vi "Derivative of intensity graph-JKI SM.vi"() -> ()   [LabVIEW 2016] (continued)
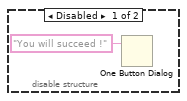
[diagram p2: hidden frame]
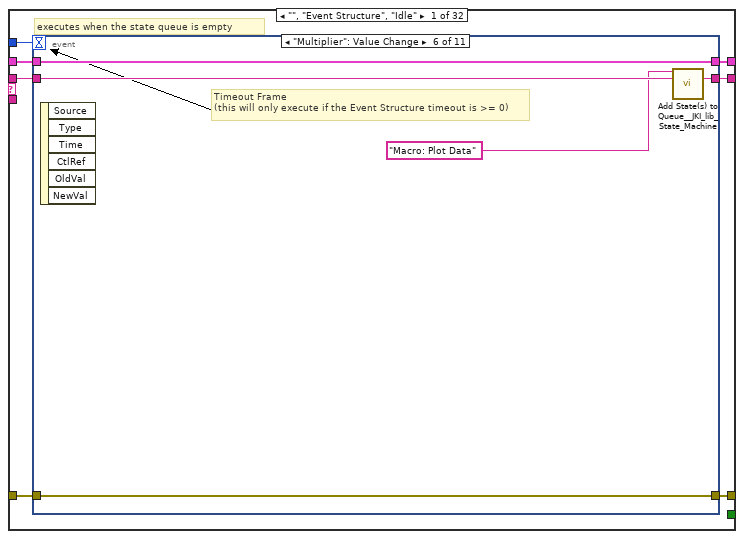
[diagram p3: hidden frame]
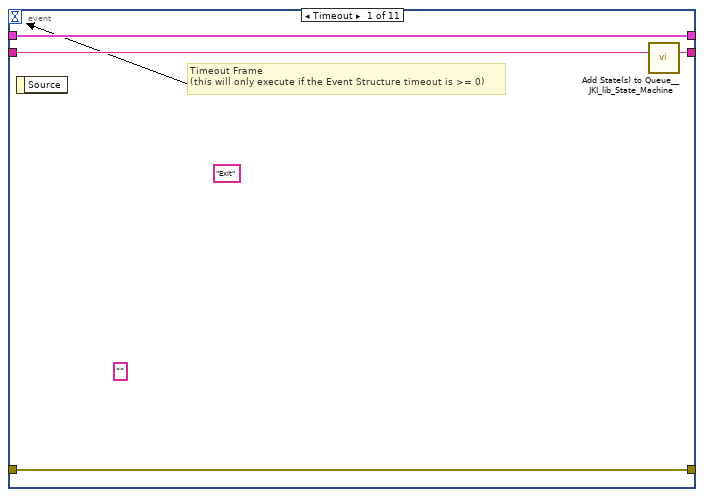
[diagram p4: hidden frame]
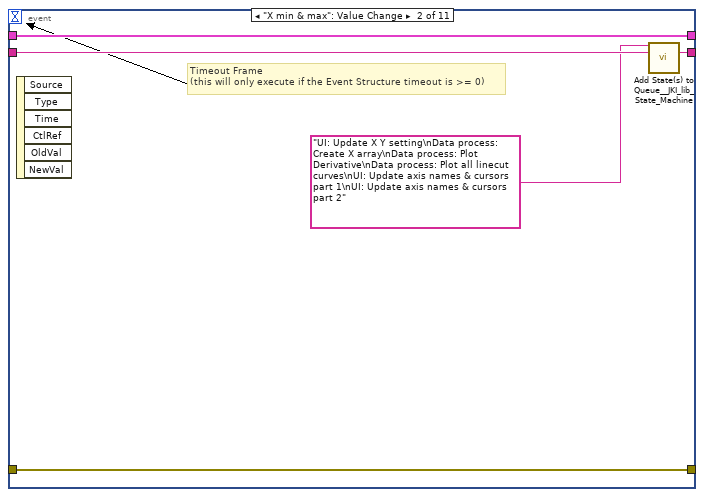
[diagram p5: hidden frame]
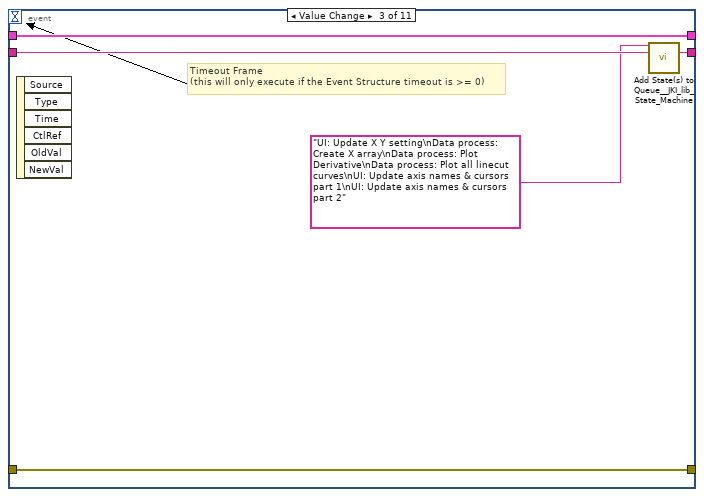
[diagram p6: hidden frame]
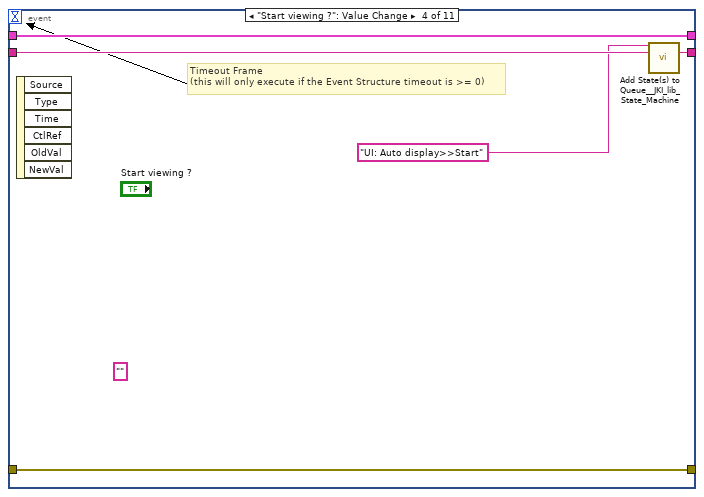
[diagram p7: hidden frame]
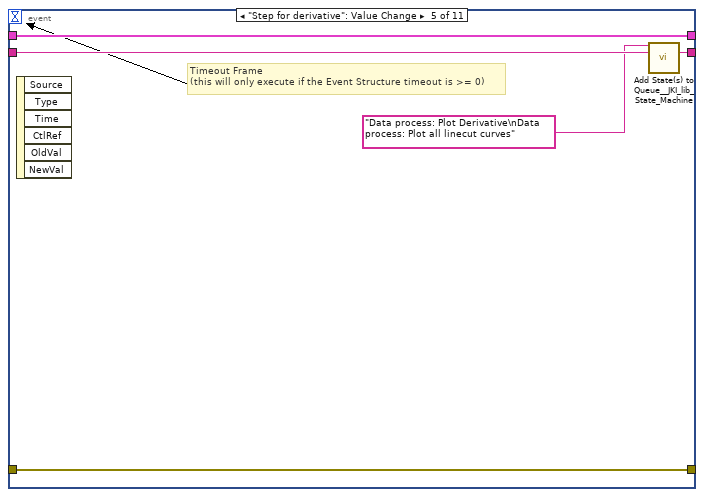
[diagram p8: hidden frame]
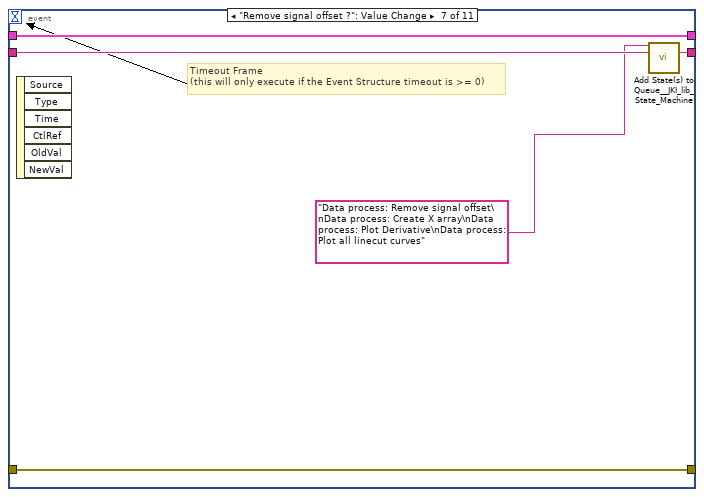
[diagram p9: hidden frame]
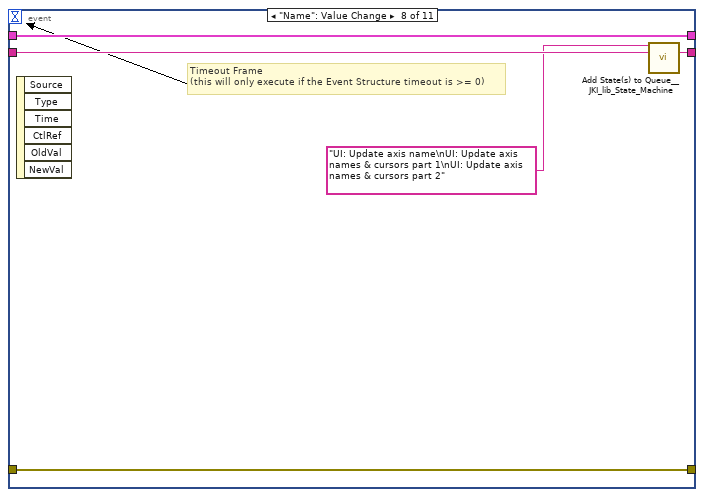
[diagram p10: hidden frame]
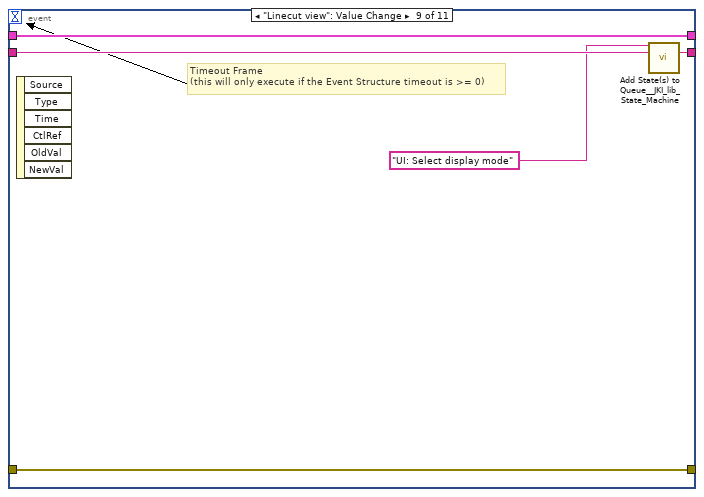
[diagram p11: hidden frame]
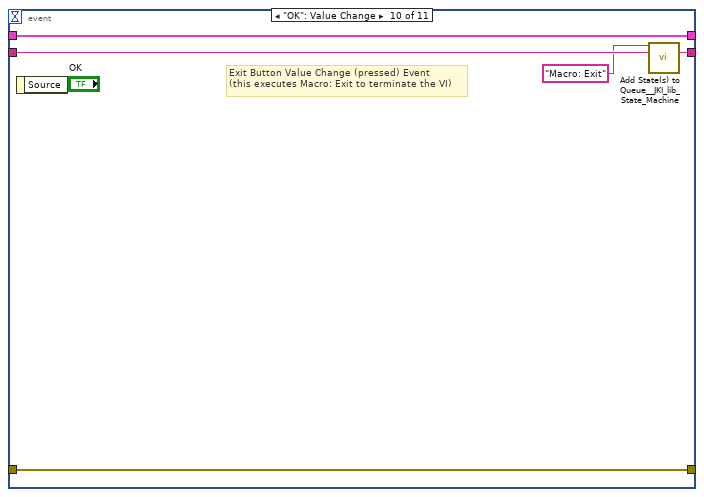
[diagram p12: hidden frame]
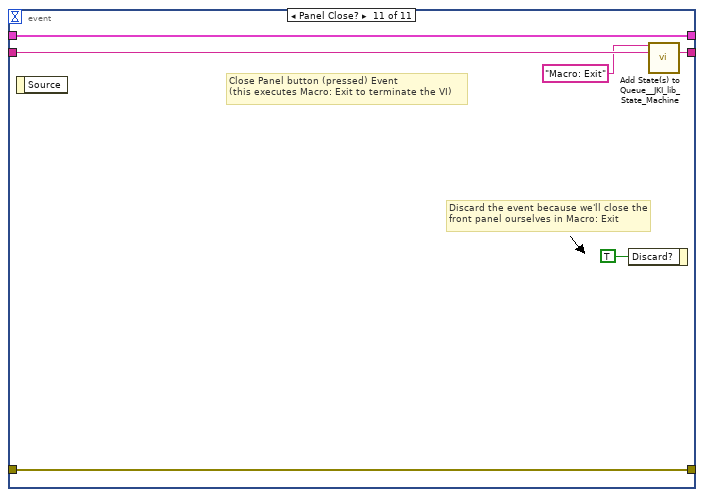
[diagram p13: hidden frame]
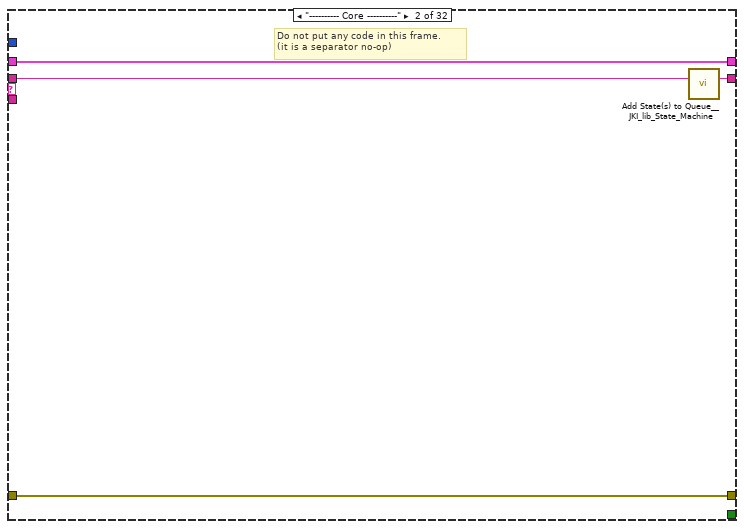
[diagram p14: hidden frame]
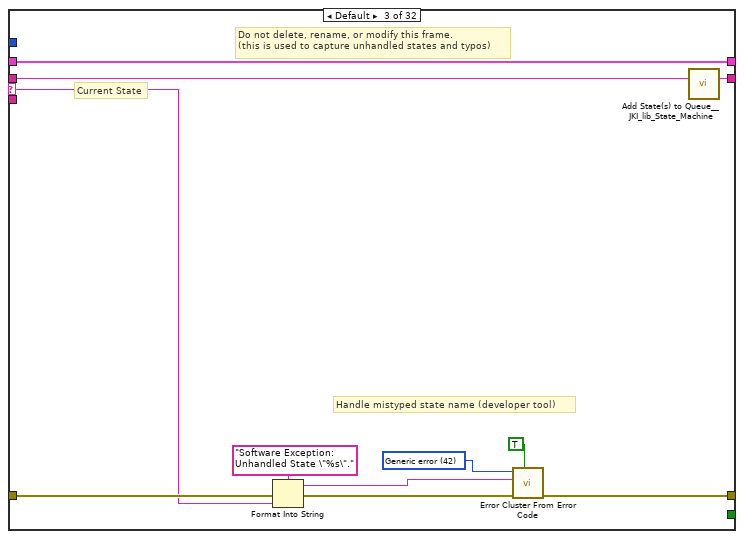
[diagram p15: hidden frame]
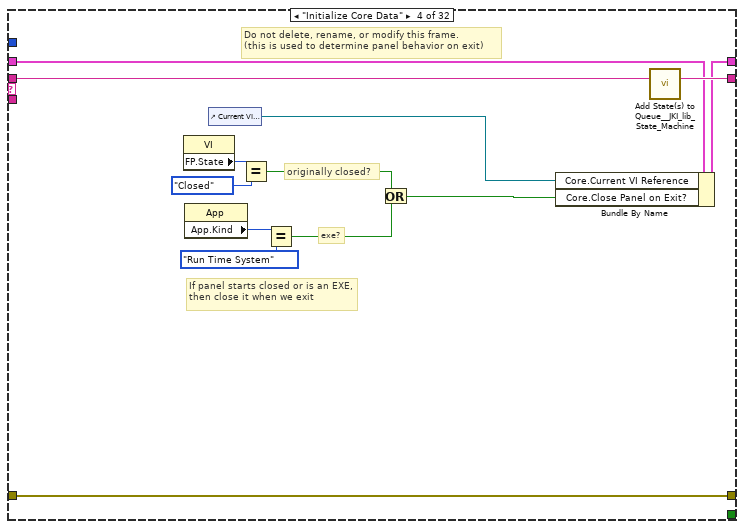
[diagram p16: hidden frame]
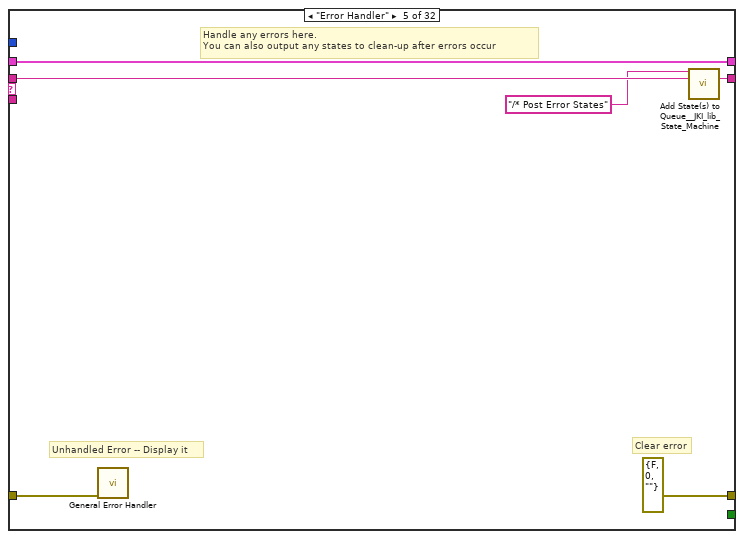
[diagram p17: hidden frame]
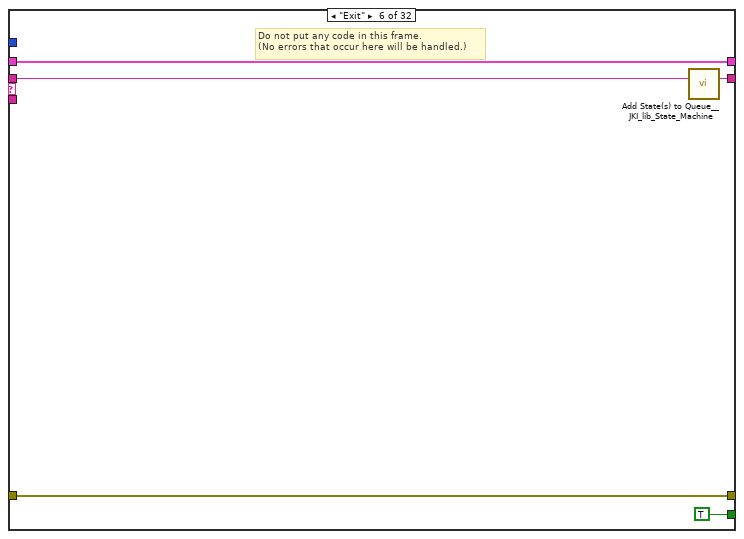
[diagram p18: hidden frame]
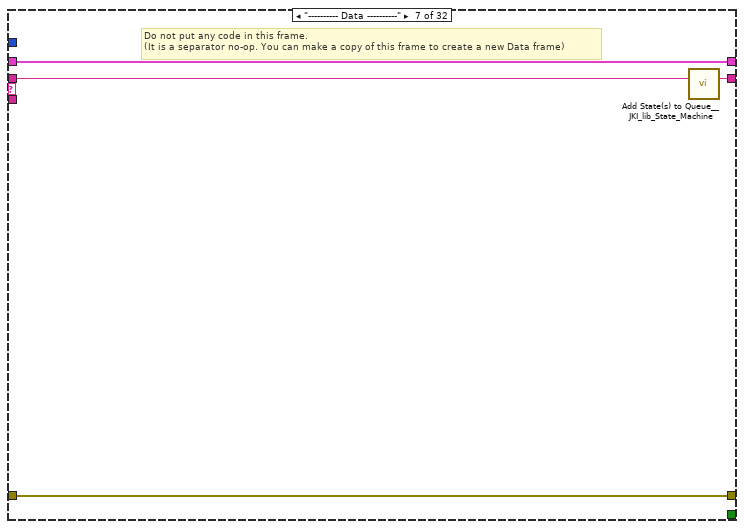
[diagram p19: hidden frame]
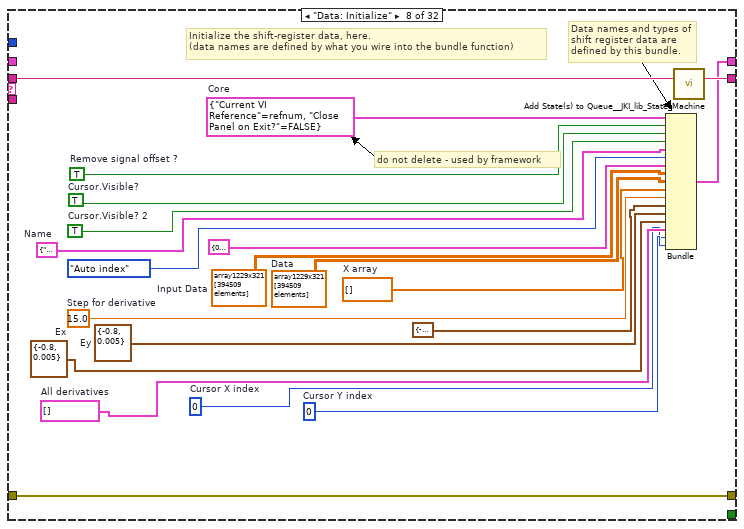
[diagram p20: hidden frame]
        # "Current State"
        # "Do not delete, rename, or modify this frame.\n(this is used to capture unhandled states and typos)"
        # "Handle mistyped state name (developer tool)"
        n30 = Format Into String(format string="Software Exception: Unhandled State \"%s\"." ("message"), error in=w85, w80) -> (resulting string=w88:string, error out=w87:errorcluster)  [unwired: 1 in]
        n31 = call <vilib>:"Error Cluster From Error Code.vi"("show call chain? (False)"=TRUE, "error in (no error)"=w87, "error message (\"\")"=w88, "error code (0)"=w89) -> ("error out"=w86:errorcluster)  [unwired: 5 in]
        n32 = call <vilib>:"Add State(s) to Queue__JKI_lib_State_Machine.vi"("State(s) in (\"\")"=w84) -> ("States Out"=w83:string)  [unwired: 14 in]
      }
      frame "Initialize Core Data" {
        # "Do not delete, rename, or modify this frame.\n(this is used to determine panel behavior on exit)"
        # "originally closed?"
        # "exe?"
        # "If panel starts closed or is an EXE, then close it when we exit"
        n33 = property class="VI"() -> ("FP.State"=w93:T5)  [unwired: 2 in, 2 out]
        n34 = property class="App"() -> ("App.Kind"=w99:T6)  [unwired: 2 in, 2 out]
        n35 = control-ref of="Current VI Reference"() -> (w94:refnum<vi>)
        n36 = Equal?(x=w93, y=T5."Closed" ("Front Panel Window:State")) -> (x = y?=w91:bool)
        n37 = Equal?(x=w99, y=T6."Run Time System" ("Application:Kind")) -> (x = y?=w97:bool)
        n38 = Or(x=w91, y=w97) -> (x .or. y?=w95:bool)
        n39 = Bundle By Name(cluster=w96, "Core.Current VI Reference"=w94, "Core.Close Panel on Exit?"=w95) -> (w101:T7)
        n40 = call <vilib>:"Add State(s) to Queue__JKI_lib_State_Machine.vi"("State(s) in (\"\")"=w103) -> ("States Out"=w102:string)  [unwired: 14 in]
      }
      frame "Error Handler" {
        # "Unhandled Error -- Display it"
        # "Handle any errors here.\nYou can also output any states to clean-up after errors occur"
        # "Clear error"
        n41 = call <vilib>:"General Error Handler.vi"("error in (no error)"=w105) -> ()  [unwired: 10 in, 5 out]
        n42 = call <vilib>:"Add State(s) to Queue__JKI_lib_State_Machine.vi"("State(s) in Front (\"\")"="/* Post Error States", "State(s) in (\"\")"=w109) -> ("States Out"=w108:string)  [unwired: 13 in]
      }
      frame "Exit" {
        # "Do not put any code in this frame.\n(No errors that occur here will be handled.)"
        n43 = call <vilib>:"Add State(s) to Queue__JKI_lib_State_Machine.vi"("State(s) in (\"\")"=w114) -> ("States Out"=w113:string)  [unwired: 14 in]
      }
      frame "---------- Data ----------" {
        # "Do not put any code in this frame.\n(It is a separator no-op. You can make a copy of this frame to create a new Data frame)"
        n44 = call <vilib>:"Add State(s) to Queue__JKI_lib_State_Machine.vi"("State(s) in (\"\")"=w118) -> ("States Out"=w117:string)  [unwired: 14 in]
      }
      frame "Data: Initialize" {
        w120 = T1 {"Offset"=-0.8, "Multiplier"=0.005}  # Ex
        w122 = 0  # Cursor Y index
        w121 = 0  # Cursor X index
        w123 = cluster{dbl[], dbl[]}[] []  # All derivatives
        w124 = dbl[] []  # X array
        w125 = dbl[][] array1229x321[394509 elements]  # Data
        w126 = T1 {"Offset"=-0.8, "Multiplier"=0.005}  # Ey
        w127 = 15.0  # Step for derivative
        w128 = dbl[][] array1229x321[394509 elements]  # Input Data
        w131 = T4 {"X"="Vsd (V)", "Y"="VsgL (V)", "Z"="I (A)", "dZ/dX"="dI/dV (S)"}  # Name
        w132 = TRUE  # Cursor.Visible? 2
        w133 = TRUE  # Cursor.Visible?
        w134 = T8 {"Current VI Reference"=refnum, "Close Panel on Exit?"=FALSE}  # Core
        w135 = TRUE  # Remove signal offset ?
        # "do not delete - used by framework"
        # "Data names and types of shift register data are defined by this bundle."
        # "Initialize the shift-register data, here.\n(data names are defined by what you wire into the bundle function)"
        n45 = Bundle("Core"=w134, "Remove signal offset ?"=w135, "Cursor.Visible?"=w133, "Cursor.Visible? 2"=w132, "Name"=w131, "Linecut view"=enum16{"Manual index", "Auto index"}."Auto index", "Signal offset to Subtract"=T3 {"X value"=0.0, "Y value"=0.0, "X for all Y values ?"=FALSE}, "Input Data"=w128, "Data"=w125, "X array"=w124, "Step for derivative"=w127, "X min & max"=cluster{"X min":dbl, "X max":dbl} {"X min"=-0.1923, "X max"=0.2993}, "Ey"=w126, "Ex"=w120, "All derivatives"=w123, "Cursor X index"=w121, "Cursor Y index"=w122) -> (w137:T7)  [unwired: 1 in]
        n46 = call <vilib>:"Add State(s) to Queue__JKI_lib_State_Machine.vi"("State(s) in (\"\")"=w139) -> ("States Out"=w138:string)  [unwired: 14 in]
      }
      frame "Data: Cleanup" {
        # "Cleanup any data and references, here.\n(this is called automatically, by the Macro: Exit)"
        n47 = Unbundle By Name(w140) -> ("Core.Current VI Reference"=w143:refnum<vi>)
        n48 = Close Reference(reference=w143, error in (no error)=w142) -> (error out=w141:errorcluster)
        n49 = call <vilib>:"Add State(s) to Queue__JKI_lib_State_Machine.vi"("State(s) in (\"\")"=w145) -> ("States Out"=w144:string)  [unwired: 14 in]
      }
      frame "---------- UI ----------" {
        # "Do not put any code in this frame.\n(It is a separator no-op. You can make a copy of this frame to create a new UI frame)"
        n50 = call <vilib>:"Add State(s) to Queue__JKI_lib_State_Machine.vi"("State(s) in (\"\")"=w149) -> ("States Out"=w148:string)  [unwired: 14 in]
      }
      frame "UI: Initialize" {
        # "Initialize the User Interface, here.\n(this is called automatically, by the Macro: Init)"
        n51 = call <vilib>:"Add State(s) to Queue__JKI_lib_State_Machine.vi"("State(s) in (\"\")"=w153) -> ("States Out"=w152:string)  [unwired: 14 in]
      }
      frame "UI: Cursor Set" {
        # "Argument"
        # "Set and Unset Cursor Busy.\n(Usage: \"UI: Cursor Set >> Busy|Idle\")"
        n52 = case shown="\"Idle\", Default" w154 {
          tunnel: w156 -> [w161 w163]
          tunnel: [w160 w162] -> w155
          frame "Idle", Default {
            n53 = call <vilib>:"Unset Busy.vi"("error in (no error)"=w161) -> ("error out"=w160:errorcluster)  [unwired: 10 in]
          }
          frame "Busy" {
            n54 = call <vilib>:"Set Busy.vi"("error in (no error)"=w163) -> ("error out"=w162:errorcluster)  [unwired: 9 in, 1 out]
          }
        }
        n55 = call <vilib>:"Add State(s) to Queue__JKI_lib_State_Machine.vi"("State(s) in (\"\")"=w159) -> ("States Out"=w158:string)  [unwired: 14 in]
      }
      frame "UI: Front Panel State" {
        # "Argument"
        # "Set Front Panel Open or Closed\n(Usage: \"UI: Front Panel State >> Open|Close\")"
        n56 = Unbundle By Name(w166) -> ("Core.Current VI Reference"=w165:refnum<vi>)
        n57 = case shown="\"Open\", \"Standard\", Default" w164 {
          tunnel: w168 -> [w176 w191 w202 w215 w228]
          tunnel: [w178 w192 w204 w217 w230] -> w167
          tunnel: w165 -> [w177 w189 w203 w216 w229]
          frame "Open", "Standard", Default {
            w171 = T5."Standard" ("State")
            n58 = property class="VI"(reference=w177, error in=w176) -> (reference out=w174:refnum<vi>, error out=w175:errorcluster, "FP.State"=w173:T5)
            n59 = Not Equal?(x=w173, y=w171) -> (x != y?=w172:bool)
            n60 = case shown="False" w172 {
              tunnel: [w182 w184] -> w178
              tunnel: w175 -> [w181 w184]
              tunnel: w174 -> [w180 _]
              tunnel: w171 -> [w179 _]
              frame True {
                n61 = invoke class="VI" method="FP.Open"(reference=w180, error in=w181, "Activate"=TRUE, "State"=w179) -> (error out=w182:errorcluster)  [unwired: 1 in, 4 out]
              }
              frame False {
              }
            }
          }
          frame "Close", "Closed" {
            n62 = property class="VI"(reference=w189, error in=w191) -> (reference out=w188:refnum<vi>, error out=w190:errorcluster, "FP.State"=w186:T5)
            n63 = Not Equal?(x=w186, y=T5."Closed" ("Front Panel Window:State")) -> (x != y?=w185:bool)
            n64 = case shown="True" w185 {
              tunnel: [w193 w196] -> w192
              tunnel: w190 -> [w193 w195]
              tunnel: w188 -> [_ w194]
              frame False {
              }
              frame True {
                n65 = invoke class="VI" method="FP.Close"(reference=w194, error in=w195) -> (error out=w196:errorcluster)  [unwired: 1 in, 2 out]
              }
            }
          }
          frame "Hidden", "Hide" {
            w197 = T5."Hidden" ("State")
            n66 = property class="VI"(reference=w203, error in=w202) -> (reference out=w200:refnum<vi>, error out=w201:errorcluster, "FP.State"=w199:T5)
            n67 = Not Equal?(x=w199, y=w197) -> (x != y?=w198:bool)
            n68 = case shown="True" w198 {
              tunnel: [w208 w209] -> w204
              tunnel: w201 -> [w207 w209]
              tunnel: w200 -> [w206 _]
              tunnel: w197 -> [w205 _]
              frame True {
                n69 = invoke class="VI" method="FP.Open"(reference=w206, error in=w207, "State"=w205) -> (error out=w208:errorcluster)  [unwired: 2 in, 4 out]
              }
              frame False {
              }
            }
          }
          frame "Minimize", "Minimized" {
            w210 = T5."Minimized" ("State")
            n70 = property class="VI"(reference=w216, error in=w215) -> (reference out=w213:refnum<vi>, error out=w214:errorcluster, "FP.State"=w212:T5)
            n71 = Not Equal?(x=w212, y=w210) -> (x != y?=w211:bool)
            n72 = case shown="True" w211 {
              tunnel: [w221 w222] -> w217
              tunnel: w214 -> [w220 w222]
              tunnel: w213 -> [w219 _]
              tunnel: w210 -> [w218 _]
              frame True {
                n73 = invoke class="VI" method="FP.Open"(reference=w219, error in=w220, "State"=w218) -> (error out=w221:errorcluster)  [unwired: 2 in, 4 out]
              }
              frame False {
              }
            }
          }
          frame "Maximize", "Maximized" {
            w223 = T5."Maximized" ("State")
            n74 = property class="VI"(reference=w229, error in=w228) -> (reference out=w226:refnum<vi>, error out=w227:errorcluster, "FP.State"=w225:T5)
            n75 = Not Equal?(x=w225, y=w223) -> (x != y?=w224:bool)
            n76 = case shown="True" w224 {
              tunnel: [w234 w235] -> w230
              tunnel: w227 -> [w233 w235]
              tunnel: w226 -> [w232 _]
              tunnel: w223 -> [w231 _]
              frame True {
                n77 = invoke class="VI" method="FP.Open"(reference=w232, error in=w233, "State"=w231) -> (error out=w234:errorcluster)  [unwired: 2 in, 4 out]
              }
              frame False {
              }
            }
          }
        }
        n78 = call <vilib>:"Add State(s) to Queue__JKI_lib_State_Machine.vi"("State(s) in (\"\")"=w170) -> ("States Out"=w169:string)  [unwired: 14 in]
      }
      frame "UI: Set background to Red" {
        # "Do not put any code in this frame.\n(It is a separator no-op. You can make a copy of this frame to create a new UI frame)"
        n79 = Unbundle By Name(w244) -> ("Core.Current VI Reference"=w243:refnum<vi>)
        n80 = property class="VI"(reference=w243) -> ("Panel"=w242:refnum<vi>)  [unwired: 1 in, 2 out]
        n81 = property class="Pnl"(reference=w242) -> (reference out=w241:refnum<vi>, error out=w239:errorcluster, "Panes[]"=w240:refnum<vi>[])  [unwired: 1 in]
        n82 = for {
          tunnel: w240 -> [w250] mode=indexing
          shift-right: [w247] -> w238
          shift-left: w239 -> [w248]
          n83 = property class="Pane"(reference=w250, error in=w248, "PaneColor"=u32 13816530) -> (error out=w247:errorcluster)  [unwired: 1 out]
        }
        n84 = Close Reference(reference=w240, error in (no error)=w238) -> (error out=w237:errorcluster)
        n85 = Close Reference(reference=w241, error in (no error)=w237) -> (error out=w236:errorcluster)
        n86 = call <vilib>:"Add State(s) to Queue__JKI_lib_State_Machine.vi"("State(s) in (\"\")"=w246) -> ("States Out"=w245:string)  [unwired: 14 in]
      }
      frame "UI: Select display mode" {
        # "Do not put any code in this frame.\n(It is a separator no-op. You can make a copy of this frame to create a new UI frame)"
        n87 = case shown="\"Auto index\"" "Linecut view" {
          tunnel: ["UI: Manual display" ("State(s) in Front (\"\")") "UI: Auto display" ("State(s) in Front (\"\")")] -> w251
          frame "Manual index", Default {
          }
          frame "Auto index" {
          }
        }
        n88 = call <vilib>:"Add State(s) to Queue__JKI_lib_State_Machine.vi"("State(s) in Front (\"\")"=w251, "State(s) in (\"\")"=w256) -> ("States Out"=w255:string)  [unwired: 13 in]
      }
      frame "UI: Update X Y setting" {
        # "Do not put any code in this frame.\n(It is a separator no-op. You can make a copy of this frame to create a new UI frame)"
        n89 = Unbundle By Name(w263) -> ("Data"=w265:dbl[][])
        n90 = Transpose 2D Array(2D array=w265) -> (transposed array=w269:dbl[][])
        n91 = Unbundle By Name("X min & max") -> ("X max"=w271:dbl, "X min"=w264:dbl)
        n92 = Array Size(array=w269) -> (size(s)=w268:i32[])
        n93 = Index Array(array=w268) -> (element #2=w267:i32)  [unwired: 2 in, 1 out]
        n94 = Subtract(x=w271, y=w264) -> (x-y=w270:dbl)
        n95 = Divide(x=w270, y=w267) -> (x/y=w266:dbl)
        n96 = Bundle By Name(cluster="Ey", "Multiplier"=w266, "Offset"=w264) -> (w260:T1)
        n97 = Bundle By Name(cluster=w263, "Ey"="Ey", "Ex"=w260, "X min & max"="X min & max") -> (w262:T7)
        n98 = call <vilib>:"Add State(s) to Queue__JKI_lib_State_Machine.vi"("State(s) in (\"\")"=w274) -> ("States Out"=w273:string)  [unwired: 14 in]
      }
      frame "UI: Update axis name" {
        # "Do not put any code in this frame.\n(It is a separator no-op. You can make a copy of this frame to create a new UI frame)"
        n99 = Bundle By Name(cluster=w277, "Name"="Name") -> (w276:T7)
        n100 = call <vilib>:"Add State(s) to Queue__JKI_lib_State_Machine.vi"("State(s) in (\"\")"=w280) -> ("States Out"=w279:string)  [unwired: 14 in]
      }
      frame "UI: Update axis names & cursors part 1" {
        # "Do not put any code in this frame.\n(It is a separator no-op. You can make a copy of this frame to create a new UI frame)"
        n101 = Unbundle By Name(w305) -> ("Name.X"=w287:string, "Name.Y"=w281:string, "Name.Z"=w291:string, "Name.dZ/dX"=w303:string, "Ex"=w292:T1, "Ey"=w297:T1, "Cursor X index"=w302:i32, "Cursor Y index"=w295:i32)
        n102 = Unbundle By Name(w297) -> ("Multiplier"=w296:dbl, "Offset"=w294:dbl)
        n103 = Unbundle By Name(w292) -> ("Multiplier"=w301:dbl, "Offset"=w300:dbl)
        n104 = Multiply(x=w302, y=w301) -> (x*y=w299:dbl)
        n105 = Multiply(x=w295, y=w296) -> (x*y=w298:dbl)
        n106 = Add(x=w300, y=w299) -> (x+y=w289:dbl)
        n107 = Add(x=w294, y=w298) -> (x+y=w284:dbl)
        n108 = Format Into String(format string="= %.1p", w284) -> (resulting string=w282:string)  [unwired: 2 in, 1 out]
        n109 = Concatenate Strings(w281, w282) -> (→"Y value (for X axis)":string)
        n110 = Format Into String(format string="= %.1p", w289) -> (resulting string=w288:string)  [unwired: 2 in, 1 out]
        n111 = Concatenate Strings(w287, w288) -> (→"X value (for Y axis)":string)
        n112 = property on="Data" class="IntGraph (strict)"("Cursor.Cursor X"=w289, "Cursor.Cursor Y"=w284, "XScale.Ofst&Mult"=w292, "YScale.Ofst&Mult"=w297, "Cursor.Visible"="Cursor.Visible ? - Data", "XScale.NameLbl.Text"=w287, "YScale.NameLbl.Text"=w281, "ZScale.NameLbl.Text"=w291) -> ()  [unwired: 2 in, 2 out]
        n113 = property on="Derivative of Data" class="IntGraph (strict)"("Cursor.Cursor X"=w289, "Cursor.Cursor Y"=w284, "XScale.Ofst&Mult"=w292, "YScale.Ofst&Mult"=w297, "Cursor.Visible"="Cursor.Visible ? - Derivative", "XScale.NameLbl.Text"=w287, "YScale.NameLbl.Text"=w281, "ZScale.NameLbl.Text"=w303) -> ()  [unwired: 2 in, 2 out]
        n114 = call <vilib>:"Add State(s) to Queue__JKI_lib_State_Machine.vi"("State(s) in (\"\")"=w308) -> ("States Out"=w307:string)  [unwired: 14 in]
      }
      frame "UI: Update axis names & cursors part 2" {
        # "Do not put any code in this frame.\n(It is a separator no-op. You can make a copy of this frame to create a new UI frame)"
        n115 = Unbundle By Name(w315) -> ("Name.X"=w309:string, "Name.Y"=w313:string, "Name.Z"=w310:string, "Name.dZ/dX"=w314:string, "Ex"=w311:T1, "Ey"=w312:T1)
        n116 = property on="All derivatives" class="XYGraph (strict)"("XScale.NameLbl.Text"=w309, "YScale.NameLbl.Text"=w314) -> ()  [unwired: 2 in, 2 out]
        n117 = property on="Linecut along X axis" class="WFGraph (strict)"("XScale.Ofst&Mult"=w311, "XScale.NameLbl.Text"=w309, "YScale.NameLbl.Text"=w310) -> ()  [unwired: 2 in, 2 out]
        n118 = property on="Linecut along Y axis" class="WFGraph (strict)"("XScale.Ofst&Mult"=w312, "XScale.NameLbl.Text"=w313, "YScale.NameLbl.Text"=w310) -> ()  [unwired: 2 in, 2 out]
        n119 = property on="Linecut of Data 2" class="WFGraph (strict)"("XScale.Ofst&Mult"=w311, "XScale.NameLbl.Text"=w309, "YScale.NameLbl.Text"=w310) -> ()  [unwired: 2 in, 2 out]
        n120 = property on="Linecut of derivative 2" class="XYGraph (strict)"("XScale.NameLbl.Text"=w309, "YScale.NameLbl.Text"=w310) -> ()  [unwired: 2 in, 2 out]
        n121 = property on="Linecut of derivative" class="XYGraph (strict)"("XScale.NameLbl.Text"=w309, "YScale.NameLbl.Text"=w310) -> ()  [unwired: 2 in, 2 out]
        n122 = call <vilib>:"Add State(s) to Queue__JKI_lib_State_Machine.vi"("State(s) in (\"\")"=w318) -> ("States Out"=w317:string)  [unwired: 14 in]
      }
      frame "UI: Manual display" {
        # "Do not put any code in this frame.\n(It is a separator no-op. You can make a copy of this frame to create a new UI frame)"
        n123 = Unbundle By Name(w325) -> ("Data"=w329:dbl[][], "All derivatives"=w321:cluster{dbl[], dbl[]}[])  [unwired: 2 out]
        n124 = Transpose 2D Array(2D array=w329) -> (transposed array=w327:dbl[][])
        n125 = Index Array(array=w327, index (col)="X index (Y axis)") -> (element=→"Linecut along Y axis":dbl[])  [unwired: 1 in]
        n126 = Index Array(array=w321, index="Y index (X axis)") -> (element=→"Linecut of derivative":cluster{dbl[], dbl[]})
        n127 = Index Array(array=w327, index (row)="Y index (X axis)") -> (element=→"Linecut along X axis":dbl[])  [unwired: 1 in]
        n128 = Bundle By Name(cluster=w325, "Cursor X index"="X index (Y axis)", "Cursor Y index"="Y index (X axis)") -> (w324:T7)
        n129 = call <vilib>:"Add State(s) to Queue__JKI_lib_State_Machine.vi"("State(s) in Front (\"\")"="UI: Update axis names & cursors part 1\nEvent Structure//check for UI change\nUI: Manual display" ("State(s) in Front (\"\")"), "State(s) in (\"\")"=w332) -> ("States Out"=w331:string)  [unwired: 13 in]
      }
      frame "UI: Auto display" {
        # "Do not put any code in this frame.\n(It is a separator no-op. You can make a copy of this frame to create a new UI frame)"
        n130 = case shown="\"Increment\"" w336 {
          tunnel: w335 -> [w344 w374 w378 w382]
          tunnel: w338 -> [w345 w377 w379 w383]
          tunnel: [w345 w377 w379 w383] -> w337
          tunnel: [w342 w373 w378 w382] -> w334
          tunnel: ["UI: Auto display>>Increment" ("State(s) in Front (\"\")") w358 _ _] -> w333
          frame "Start" {
            n131 = Bundle By Name(cluster=w344, "Cursor Y index"=0 ("Cursor X index")) -> (w342:T7)
          }
          frame "Increment" {
            n132 = Unbundle By Name(w374) -> ("Cursor Y index"=w350:i32, "Data"=w369:dbl[][], "All derivatives"=w371:cluster{dbl[], dbl[]}[], "Name.Y"=w346:string, "Ey"=w352:T1)
            n133 = Wait (ms)(milliseconds to wait="Wait between index") -> ()  [unwired: 1 out]
            n134 = Array Size(array=w369) -> (size(s)=w368:i32[])
            n135 = Unbundle By Name(w352) -> ("Multiplier"=w349:dbl, "Offset"=w351:dbl)
            n136 = Index Array(array=w369, index (row)=w350) -> (element=→"Linecut of Data 2":dbl[])  [unwired: 1 in]
            n137 = Add(x=w350, y="Decimate index") -> (x+y=w367:i32)
            n138 = Index Array(array=w371, index=w350) -> (element=→"Linecut of derivative 2":cluster{dbl[], dbl[]})
            n139 = Index Array(array=w368) -> (element #2=w365:i32)  [unwired: 2 in, 1 out]
            n140 = Quotient & Remainder(x=w367, y=w365) -> (x-y*floor(x/y)=w366:i32)  [unwired: 1 out]
            n141 = Multiply(x=w350, y=w349) -> (x*y=w348:dbl)
            n142 = Bundle By Name(cluster=w374, "Cursor Y index"=w366) -> (w373:T7)
            n143 = Add(x=w348, y=w351) -> (x+y=w347:dbl)
            n144 = Format Into String(format string="= %.1p", w347) -> (resulting string=w355:string)  [unwired: 2 in, 1 out]
            n145 = Concatenate Strings(w346, w355) -> (→"Y value":string)
            n146 = Select(t="UI: Auto display>>Pause\nUI: Auto display>>Increment" ("message"), s="Pause viewing ?", f="UI: Auto display>>Increment" ("message")) -> (s? t:f=w359:string)
            n147 = Select(t="" ("message"), s="stop viewing ?", f=w359) -> (s? t:f=w356:string)
            n148 = call <vilib>:"Add State(s) to Queue__JKI_lib_State_Machine.vi"("State(s) in Front (\"\")"="UI: Update axis names & cursors part 1\nUI: Update axis names & cursors part 2\n//Event Structure//Check UI changes" ("message"), "State(s) in (\"\")"=w356) -> ("States Out"=w358:string)  [unwired: 13 in]
          }
          frame "Pause", Default {
            n149 = while {
              stop <- w380 continue-if-true
              n150 = local read "Pause viewing ?"() -> (w380:bool)
              n151 = Wait (ms)(milliseconds to wait=u32 10) -> ()  [unwired: 1 out]
            }
          }
          frame "Stop" {
          }
        }
        n152 = call <vilib>:"Add State(s) to Queue__JKI_lib_State_Machine.vi"("State(s) in Front (\"\")"=w333, "State(s) in (\"\")"=w340) -> ("States Out"=w339:string)  [unwired: 13 in]
      }
      frame "---------- Macro ----------" {
        # "Do not put any code in this frame.\n(It is a separator no-op. You can make a copy of this frame to create a new Macro frame)"
        n153 = call <vilib>:"Add State(s) to Queue__JKI_lib_State_Machine.vi"("State(s) in (\"\")"=w387) -> ("States Out"=w386:string)  [unwired: 14 in]
      }
      frame "Macro: Plot Data" {
        # "Do not put any code in this frame.\n(It is a separator no-op. You can make a copy of this frame to create a new Macro frame)"
        n154 = call <vilib>:"Add State(s) to Queue__JKI_lib_State_Machine.vi"("State(s) in Front (\"\")"="Data process: Input and initialize data\nUI: Update X Y setting\nData process: Remove signal offset\nData process: Create X array\nData process: Plot Derivative\nData process: Plot all linecut curves\nUI: Update axis name\nUI: Update axis names & cursors part 1\nUI: Update axis names & cursors part 2\nUI: Select display mode" ("State(s) in Front (\"\")"), "State(s) in (\"\")"=w392) -> ("States Out"=w391:string)  [unwired: 13 in]
      }
      frame "Macro: Initialize" {
        # "Initialization Macro\n(This is called once, when the VI starts)"
        n155 = call <vilib>:"Add State(s) to Queue__JKI_lib_State_Machine.vi"("State(s) in Front (\"\")"="Data: Initialize\nInitialize Core Data\nUI: Initialize\nUI: Front Panel State >> Open\nUI: Set background to Red\nMacro: Plot Data", "State(s) in (\"\")"=w397) -> ("States Out"=w396:string)  [unwired: 13 in]
      }
      frame "Macro: Exit" {
        # "Exit Macro\n(This is called once, when the VI exits)"
        n156 = Unbundle By Name(w404) -> ("Core.Close Panel on Exit?"=w403:bool)
        n157 = Select(t="UI: Front Panel State >> Close", s=w403, f="") -> (s? t:f=w400:string)
        n158 = call <vilib>:"Add State(s) to Queue__JKI_lib_State_Machine.vi"("State(s) in (\"\")"=w400, "State(s) at Back (\"\")"="Data: Cleanup\nExit") -> ("States Out"=w398:string)  [unwired: 13 in]
        n159 = call <vilib>:"Add State(s) to Queue__JKI_lib_State_Machine.vi"("State(s) in Front (\"\")"=w398, "State(s) in (\"\")"=w407) -> ("States Out"=w406:string)  [unwired: 13 in]
      }
      frame "---------- Data process ----------" {
        # "Template Separator\n(You can make a copy of, or modify, this frame)"
        n160 = call <vilib>:"Add State(s) to Queue__JKI_lib_State_Machine.vi"("State(s) in (\"\")"=w411) -> ("States Out"=w410:string)  [unwired: 14 in]
      }
      frame "Data process: Input and initialize data" {
        # "Template Separator\n(You can make a copy of, or modify, this frame)"
        n161 = Multiply(x="Input Data", y="Multiplier") -> (x*y=w412:dbl[][])
        n162 = Bundle By Name(cluster=w416, "Input Data"=w412) -> (w415:T7)
        n163 = call <vilib>:"Add State(s) to Queue__JKI_lib_State_Machine.vi"("State(s) in (\"\")"=w419) -> ("States Out"=w418:string)  [unwired: 14 in]
      }
      frame "Data process: Remove signal offset" {
        # "Template Separator\n(You can make a copy of, or modify, this frame)"
        n164 = Unbundle By Name(w432) -> ("Input Data"=w422:dbl[][], "X min & max"=w426:cluster{"X min":dbl, "X max":dbl}, "Ey"=w425:T1)
        n165 = call "Remove signal offset - Intensity graph.vi"("Y Scale.Offset and Multiplier"=w425, "X min & max"=w426, "Current offset to Subtract"="Signal offset to Subtract", "Data"=w422) -> ("element"=w424:dbl, "Data 2"=w421:dbl[][])  [unwired: 6 in]
        n166 = Select(t=w421, s="Remove signal offset ?", f=w422) -> (s? t:f=w420:dbl[][])
        "Data" <- w420
        n167 = Format Into String(format string="%.3p", w424) -> (resulting string=w429:string)  [unwired: 2 in, 1 out]
        n168 = Bundle By Name(cluster=w432, "Data"=w420) -> (w431:T7)
        n169 = Concatenate Strings(w429, "A" ("string")) -> (→"Signal offset":string)
        n170 = call <vilib>:"Add State(s) to Queue__JKI_lib_State_Machine.vi"("State(s) in (\"\")"=w436) -> ("States Out"=w435:string)  [unwired: 14 in]
      }
      frame "Data process: Create X array" {
        # "Template Separator\n(You can make a copy of, or modify, this frame)"
        n171 = Unbundle By Name(w438) -> ("Data"=w447:dbl[][], "Ey.Multiplier"=w444:dbl, "Ey.Offset"=w440:dbl)
        n172 = Subtract(x=w444, y=w440) -> (x-y=w443:dbl)
        n173 = Transpose 2D Array(2D array=w447) -> (transposed array=w446:dbl[][])
        n174 = Array Size(array=w446) -> (size(s)=w445:i32[])
        n175 = Index Array(array=w445) -> (element #2=w442:i32)  [unwired: 2 in, 1 out]
        n176 = Divide(x=w443, y=w442) -> (x/y=w441:dbl)
        n177 = for {
          N: w442 -> [_]
          tunnel: [w453] -> w439 mode=indexing
          tunnel: w441 -> [w452]
          tunnel: w440 -> [w451]
          i -> [w455]
          # "Create X array"
          n178 = Multiply(x=w452, y=w455) -> (x*y=w454:dbl)
          n179 = Add(x=w451, y=w454) -> (x+y=w453:dbl)
        }
        n180 = Bundle By Name(cluster=w438, "X array"=w439) -> (w437:T7)
        n181 = call <vilib>:"Add State(s) to Queue__JKI_lib_State_Machine.vi"("State(s) in (\"\")"=w450) -> ("States Out"=w449:string)  [unwired: 14 in]
      }
      frame "Data process: Plot Derivative" {
        # "Template Separator\n(You can make a copy of, or modify, this frame)"
        n182 = Unbundle By Name(w459) -> ("Data"=w464:dbl[][], "X array"=w461:dbl[])
        n183 = Transpose 2D Array(2D array=w464) -> (transposed array=w463:dbl[][])
        n184 = for {
          tunnel: [w475] -> w460 mode=indexing
          tunnel: w461 -> [w471]
          tunnel: w463 -> [w472] mode=indexing
          tunnel: [w473] -> w457 mode=indexing
          tunnel: "Step for derivative" -> [w470]
          shift-right: [w469] -> w465
          shift-left: w466 -> [w469]
          # "dz/dx vs x"
          # "After getting slopes for every section, it plots slope VS middle x of every section."
          # "It do linear fit of the small section you define in Numeric and collect all the slopes at different X"
          n185 = Array Size(array=w471) -> (size(s)=w474:i32)
          n186 = Subtract(x=w474, y=w470) -> (x-y=w477:dbl)
          n187 = Divide(x=w470, y=2.0) -> (x/y=w478:dbl)
          n188 = Increment(x=w477) -> (x+1=w480:dbl)
          n189 = for {
            N: w480 -> [_]
            tunnel: w471 -> [w487]
            tunnel: w472 -> [w486]
            tunnel: w470 -> [w484]
            tunnel: [w483] -> w473 mode=indexing
            i -> [w485]
            n190 = Array Subset(array=w487, index=w485, length=w484) -> (w481:dbl[])
            n191 = Array Subset(array=w486, index=w485, length=w484) -> (w482:dbl[])
            n192 = call <vilib>:"Linear Fit.vi"("Y"=w482, "X"=w481) -> ("slope"=w483:dbl)  [unwired: 9 in, 4 out]
          }
          n193 = Array Subset(array=w471, index=w478, length=w477) -> (w476:dbl[])
          n194 = Bundle(w476, w473) -> (w475:cluster{dbl[], dbl[]})  [unwired: 1 in]
        }
        n195 = Bundle By Name(cluster=w459, "All derivatives"=w460) -> (w458:T7)
        n196 = Transpose 2D Array(2D array=w457) -> (transposed array=→"Derivative of Data":dbl[][])
        n197 = call <vilib>:"Add State(s) to Queue__JKI_lib_State_Machine.vi"("State(s) in (\"\")"=w468) -> ("States Out"=w467:string)  [unwired: 14 in]
      }
      frame "Data process: Plot all linecut curves" {
        # "Template Separator\n(You can make a copy of, or modify, this frame)"
        n198 = Unbundle By Name(w495) -> ("Data"=w494:dbl[][], "X array"=w492:dbl[], "All derivatives"=→"All derivatives":cluster{dbl[], dbl[]}[])
        n199 = Transpose 2D Array(2D array=w494) -> (transposed array=w493:dbl[][])
        n200 = for {
          tunnel: w493 -> [w501] mode=indexing
          tunnel: w492 -> [w500]
          tunnel: [w499] -> w491 mode=indexing
          shift-right: [w498] -> w489
          shift-left: w490 -> [w498]
          n201 = Bundle("X array"=w500, w501) -> (w499:cluster{"X array":dbl[], dbl[]})  [unwired: 1 in]
        }
        "All Data" <- w491
        n202 = call <vilib>:"Add State(s) to Queue__JKI_lib_State_Machine.vi"("State(s) in (\"\")"=w497) -> ("States Out"=w496:string)  [unwired: 14 in]
      }
      frame "---------- New Category ----------" {
        # "Template Separator\n(You can make a copy of, or modify, this frame)"
        n203 = call <vilib>:"Add State(s) to Queue__JKI_lib_State_Machine.vi"("State(s) in (\"\")"=w505) -> ("States Out"=w504:string)  [unwired: 14 in]
      }
    }
  }
  n204 = disable-structure shown="Enabled" {
    frame Disabled {
      n205 = One Button Dialog(message="You will succeed !") -> ()  [unwired: 1 in, 1 out]
    }
    frame Enabled {
    }
  }
